vi "MartinsDCtest.vi"() -> ()   [LabVIEW 2011] (continued)
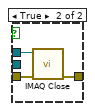
[diagram p3: hidden frame]
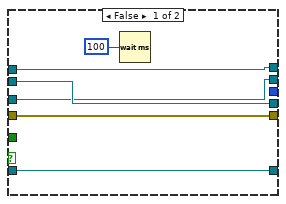
[diagram p5: hidden frame]
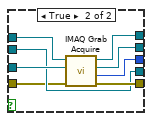
[diagram p6: hidden frame]
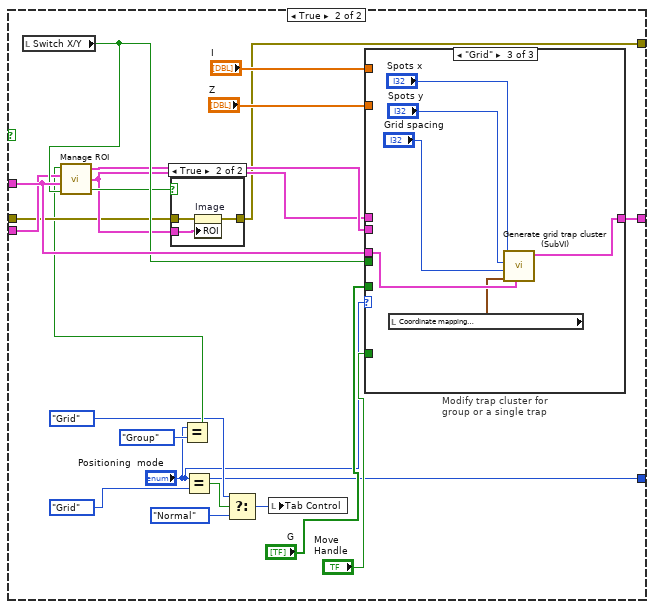
[diagram p11: hidden frame]
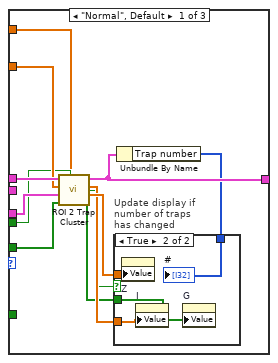
[diagram p13: hidden frame]
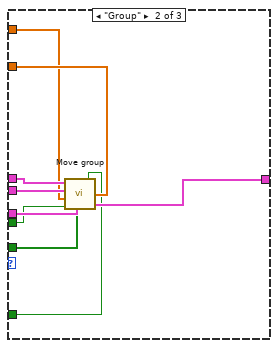
[diagram p15: hidden frame]
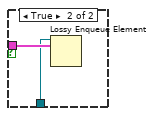
[diagram p17: hidden frame]
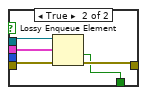
[diagram p19: hidden frame]
        }
      }
      "Step number" <- w131
    }
    n78 = local read "Stop program"() -> (w130:bool)
  }
  n79 = while "User input and events loop" {
    tunnel: w54 -> [w291]
    tunnel: w17 -> [w280]
    tunnel: w19 -> [w279]
    tunnel: w20 -> [w278]
    tunnel: [w277] -> w29
    tunnel: w28 -> [w276]
    tunnel: [w275] -> w27
    stop <- w283 stop-if-true
    w288 = u32 8 items=["Zoom Tool"=8, "Selection Tool"=0, "Pan Tool"=9, "Point Tool"=1, "Line Tool"=2, "Rectangle Tool"=3, "Rotated Rectangle Tool"=12, "Polyline Tool"=10, "Polygon Tool"=5, "Freehand Tool"=11, "Closed Freehand Tool"=6, "Ellipse Tool"=4, "Annulus Tool"=7] ("Current ROI Tool")
    w285 = T10 [enum."LCONTROL"] items=["0", "1", "2", "3", "4", "5", "6", "7", "8", "9", "A", "B", "C", "D", "E", "F", "G", "H", "I", "J", "K", "L", "M", "N", "O", "P", "Q", "R", "S", "T", "U", "V", "W", "X", "Y", "Z", "F1", "F2", "F3", "F4", "F5", "F6", "F7", "F8", "F9", "F10", "F11", "F12", "F13", "F14", "F15", "ADD", "BACK", "BACKSLASH", "CAPITAL", "COMMA", "DECIMAL", "DELETE", "DIVIDE", "DOWN", "END", "EQUALS", "ESCAPE", "GRAVE (`)", "HOME", "INSERT", "LBRACKET", "LCONTROL", "LEFT", "L ALT", "LSHIFT", "LWIN", "MINUS", "MULTIPLY", "NEXT", "NUMLOCK", "NUMPAD_0", "NUMPAD_1", "NUMPAD_2", "NUMPAD_3", "NUMPAD_4", "NUMPAD_5", "NUMPAD_6", "NUMPAD_7", "NUMPAD_8", "NUMPAD_9", "PAUSE", "PERIOD", "PRIOR (PG UP)", "RBRACKET", "RCONTROL", "RETURN", "RIGHT", "R ALT", "RSHIFT", "RWIN", "SCROLL", "SEMICOLON", "SLASH", "SPACE", "SUBTRACT", "TAB", "UP", "ENTER (num pad)", "' (quote)"] ("keys pressed")
    n80 = call-poly <vilib>:"Acquire Input Data.vi"("device ID"=w291, "error in (no error)"=w276) -> ("device ID"=w277:refnum<k1>, "keys pressed"=w284:T10, "error out"=w275:errorcluster)  [unwired: 15 out]
    n81 = property on="Image" class="ImageControl"() -> ("Current ROI Tool"=w287:u32)  [unwired: 2 in, 2 out]
    n82 = Equal?(x=w284, y=w285) -> (x = y?=w286:bool[])
    n83 = Not Equal?(x=w287, y=w288) -> (x != y?=w289:bool)
    n84 = Or Array Elements(Boolean array=w286) -> (logical OR=w290:bool)
    n85 = case shown="True" w289 {
      tunnel: w290 -> [_ w312]
      frame False {
      }
      frame True {
        n86 = case shown="False" w312 {
          frame False {
            w313 = u32 0 items=["Zoom Tool"=8, "Selection Tool"=0, "Pan Tool"=9, "Point Tool"=1, "Line Tool"=2, "Rectangle Tool"=3, "Rotated Rectangle Tool"=12, "Polyline Tool"=10, "Polygon Tool"=5, "Freehand Tool"=11, "Closed Freehand Tool"=6, "Ellipse Tool"=4, "Annulus Tool"=7] ("Current ROI Tool")
            n87 = property on="Image" class="ImageControl"("Current ROI Tool"=w313) -> ()  [unwired: 2 in, 2 out]
          }
          frame True {
            w314 = u32 1 items=["Zoom Tool"=8, "Selection Tool"=0, "Pan Tool"=9, "Point Tool"=1, "Line Tool"=2, "Rectangle Tool"=3, "Rotated Rectangle Tool"=12, "Polyline Tool"=10, "Polygon Tool"=5, "Freehand Tool"=11, "Closed Freehand Tool"=6, "Ellipse Tool"=4, "Annulus Tool"=7] ("Current ROI Tool")
            n88 = property on="Image" class="ImageControl"("Current ROI Tool"=w314) -> ()  [unwired: 2 in, 2 out]
          }
        }
      }
    }
    n89 = Wait (ms)(milliseconds to wait=u32 50) -> ()  [unwired: 1 out]
    n90 = case shown="False" "View Licence" {
      frame False {
      }
      frame True {
        n91 = call "View license.vi"() -> ()  [unwired: 1 in]
      }
    }
    n92 = event shown="[4] \"Image\", \"Positioning  mode\", \"Z\", \"I\", \"Coordinate mapping \n(IMAQ to SLM)\": Mouse Down;  Key Up" {
      selector: _ -> [_ _ _ _ _ _]
      dyn-events: _ -> [_ _ _ _ _ _]
      timeout: 0 -> [_ _ _ _ _ _]
      tunnel: w280 -> [_ _ w302 _ _ _]
      tunnel: w279 -> [_ _ w301 _ _ _]
      tunnel: w278 -> [_ _ w305 _ _ _]
      event Timeout {
        n93 = event-data() -> ()  [unwired: 1 in, 2 out]
      }
      event "Display hologram\nand computed \nimage plane": Value Change {
        n94 = event-data() -> ("NewVal"=w293:bool)  [unwired: 1 in, 4 out]
        n95 = property on="Current trap pos" class="Clust (strict)"("Visible"=w293) -> ()  [unwired: 2 in, 2 out]
        n96 = property on="Displayed Hologram" class="IntGraph (strict)"("Visible"=w293) -> ()  [unwired: 2 in, 2 out]
        n97 = property on="Calculated image plane" class="IntGraph (strict)"("Visible"=w293) -> ()  [unwired: 2 in, 2 out]
        n98 = property on="Property Node" class="VI"() -> ("Front Panel.WinBounds"=w300:T11)  [unwired: 2 in, 2 out]
        n99 = Unbundle By Name(w300) -> ("right"=w299:i16, "left"=w298:i16)
        n100 = Subtract(x=w299, y=w298) -> (x-y=w297:i16)
        n101 = Select(t=i16 500 ("x-y"), s=w293, f=i16 196 ("x-y")) -> (s? t:f=w292:i16)
        n102 = Subtract(x=w297, y=w292) -> (x-y=w296:i16)
        n103 = property on="Splitter" class="Splitter"("Position"=w296) -> ()  [unwired: 2 in, 2 out]
      }
      event "Create path": Value Change {
        n104 = event-data() -> ()  [unwired: 1 in, 5 out]
        n105 = property on="follow path" class="Bool (strict)"("Value"=FALSE) -> ()  [unwired: 2 in, 2 out]
        n106 = Flush Queue "Flush path \nwaypt queue"(queue=w301) -> ()  [unwired: 1 in, 3 out]
        n107 = Preview Queue Element(queue=w302) -> (element=w303:T3, error out=w306:errorcluster)  [unwired: 2 in, 2 out]
        n108 = Flush Queue "Flush path queue"(queue=w305) -> (queue out=w304:refnum<queue>)  [unwired: 1 in, 2 out]
        n109 = Enqueue Element "Enqueue current \ntrap pos in path"(queue=w304, element=w303) -> ()  [unwired: 2 in, 3 out]
        n110 = Enqueue Element "Enqueue current \ntrap pos in path \nwaypts"(queue=w301, element=w303, error in (no error)=w306) -> ()  [unwired: 1 in, 3 out]
      }
      event "cancel path": Value Change {
        n111 = event-data() -> ()  [unwired: 1 in, 5 out]
        n112 = local write "Create path"(FALSE ("Visible")) -> ()
      }
      event "Image", "Positioning  mode", "Z", "I", "Coordinate mapping \n(IMAQ to SLM)": Mouse Down; Key Up {
        n113 = event-data() -> ()  [unwired: 1 in, 3 out]
        n114 = local write "Updating trap cluster"(TRUE ("Update trap positions")) -> ()
      }
      event "Positioning  mode", "Z", "I", "Image", "Coordinate mapping \n(IMAQ to SLM)": Mouse Up {
        n115 = event-data() -> ()  [unwired: 1 in, 7 out]
        n116 = flat-sequence {
          frame #0 {
            n117 = Wait (ms)(milliseconds to wait=u32 100) -> ()  [unwired: 1 out]
          }
          frame #1 {
            n118 = local write "Updating trap cluster"(FALSE ("Update trap positions")) -> ()
          }
        }
      }
    }
    n119 = local read "Stop program"() -> (w283:bool)
  }
  n120 = while "Image acquisition loop" {
    tunnel: w4 -> [w324]
    tunnel: w6 -> [w340]
    tunnel: w8 -> [w339]
    tunnel: [w338] -> w53
    tunnel: [w320] -> w52
    tunnel: w51 -> [w334]
    tunnel: w49 -> [w326]
    shift-right: ["ROI size"] -> _
    shift-left: _ -> [_]
    tunnel: w46 -> [w325]
    tunnel: [w334] -> w44
    tunnel: [w321] -> w43
    tunnel: [w333] -> w42
    tunnel: w7 -> [w332]
    tunnel: w3 -> [w331]
    tunnel: w17 -> [w330]
    tunnel: w20 -> [w329]
    tunnel: w5 -> [w327]
    tunnel: w1 -> [w315]
    stop <- w337 stop-if-true
    n121 = Flush Queue(queue=w325) -> ()  [unwired: 1 in, 3 out]
    n122 = Flush Queue(queue=w326) -> ()  [unwired: 1 in, 3 out]
    n123 = Preview Queue Element(queue=w330, timeout in ms (-1)=10 ("f")) -> (element=w319:T3)  [unwired: 1 in, 3 out]
    n124 = Get Queue Status(queue=w329, return elements? (F)="Display path") -> (elements=w322:T3[])  [unwired: 1 in, 7 out]
    n125 = call <vilib>:"Acquire Semaphore.vi"("semaphore"=w315) -> ("semaphore out"=w317:T9)  [unwired: 4 in, 2 out]
    n126 = case shown="True" w324 {
      tunnel: w340 -> [w345 w357]
      tunnel: w339 -> [w344 w356]
      tunnel: [w344 w355] -> w338
      tunnel: [w343 w354] -> w320
      tunnel: [w345 w353] -> w321
      tunnel: [w346 w352] -> w333
      tunnel: w332 -> [w346 w351]
      tunnel: w331 -> [_ w350]
      tunnel: w327 -> [w343 w349]
      tunnel: [_ w348] -> _
      tunnel: w317 -> [w341 w347]
      tunnel: [w341 w347] -> w316
      frame False {
        n127 = Wait (ms)(milliseconds to wait=u32 100) -> ()  [unwired: 1 out]
      }
      frame True {
        n128 = case shown="True" w350 {
          tunnel: w357 -> [w365 w373]
          tunnel: [w363 w372] -> w355
          tunnel: [w362 w371] -> w354
          tunnel: w356 -> [w363 w370]
          tunnel: [w364 w369] -> w353
          tunnel: [w359 w368] -> w348
          tunnel: [w361 w367] -> w352
          tunnel: w351 -> [w360 w367]
          tunnel: w349 -> [w358 w366]
          frame False {
            n129 = call <vilib>:"IMAQdx Grab.vi"("error in"=w358, "Image In"=w365, "Session In"=w360) -> ("error out"=w362:errorcluster, "Buffer Number Out"=w359:u32, "Image Out"=w364:T2, "Session Out"=w361:T7)  [unwired: 5 in]
          }
          frame True {
            n130 = call <vilib>:"IMAQ Grab Acquire.vi"("error in (no error)"=w366, "Image In"=w373, "IMAQ Session In"=w370) -> ("error out"=w371:errorcluster, "Acquired Buffer Number"=w368:u32, "Image Out"=w369:T2, "IMAQ Session Out"=w372:refnum<k11>)  [unwired: 1 in, 4 out]
          }
        }
      }
    }
    n131 = call "Create trap overlay.vi"("Current trap cluster"=w319, "Image in"=w321, "ROI size"="ROI size", "Switch X/Y"="Switch X/Y", "Path"=w322) -> ()  [unwired: 1 out]
    n132 = case shown="True" "Show image" {
      tunnel: w321 -> [_ w374]
      frame False {
      }
      frame True {
        "Image" <- w374
      }
    }
    n133 = call <vilib>:"Release Semaphore.vi"("semaphore"=w316) -> ()  [unwired: 5 in, 2 out]
    n134 = local read "Stop program"() -> (w337:bool)
  }
  n135 = while "Trap position loop" {
    tunnel: w19 -> [w386]
    tunnel: w20 -> [w383]
    shift-right: [w385] -> _
    shift-left: w16 -> [w378]
    tunnel: w18 -> [w384]
    tunnel: w17 -> [w381]
    tunnel: [w380] -> w35
    tunnel: w21 -> [w377]
    tunnel: [w375] -> w33
    stop <- "Stop program" stop-if-true
    n136 = property on="Image" class="ImageControl"(error in=w377) -> (error out=w376:errorcluster, "ROI"=w380:T1)  [unwired: 1 in, 1 out]
    n137 = case shown="False" "Run calibration" {
      selector: "Run calibration" -> [_ w582]
      tunnel: w386 -> [w411 _]
      tunnel: w378 -> [w410 w581]
      tunnel: [w390 w581] -> w385
      tunnel: w384 -> [w401 w591]
      tunnel: w383 -> [w399 _]
      tunnel: w381 -> [w396 _]
      tunnel: w380 -> [w395 w590]
      tunnel: w376 -> [w394 w586]
      tunnel: [w392 w583] -> w375
      frame False {
        n138 = case "Update trap cluster" shown="False" "Updating trap cluster" {
          tunnel: w410 -> [w413 w434]
          tunnel: [w413 w427] -> w402
          tunnel: w395 -> [_ w425]
          tunnel: w394 -> [w412 w424]
          tunnel: [w412 w423] -> w393
          tunnel: [_ "Positioning  mode"] -> w387
          frame False {
          }
          frame True {
            n139 = local read "Switch X/Y"() -> (w433:bool)
            n140 = Equal?(x="Positioning  mode", y=enum16{"Normal", "Group", "Grid"}."Group") -> (x = y?=w421:bool)
            n141 = call "Manage ROI.vi"("Switch X/Y"=w433, "Trap cluster in"=w434, "ROI in"=w425, "Group traps"=w421) -> ("Replace ROI"=w432:bool, "ROI out"=w426:T1, "Previous ROI out"=w431:T1)
            n142 = case shown="True" w432 {
              tunnel: w426 -> [_ w438]
              tunnel: w424 -> [w435 w437]
              tunnel: [w435 w436] -> w423
              frame False {
              }
              frame True {
                n143 = property on="Image" class="ImageControl"(error in=w437, "ROI"=w438) -> (error out=w436:errorcluster)  [unwired: 1 in, 1 out]
              }
            }
            n144 = Equal?(x="Positioning  mode", y=enum16{"Normal", "Group", "Grid"}."Grid") -> (x = y?=w419:bool)
            n145 = Select(t=enum32{"Normal", "Grid"}."Grid", s=w419, f=enum32{"Normal", "Grid"}."Normal" ("Tab Control")) -> (s? t:f=w416:enum32{"Normal", "Grid"})
            n146 = local write "Tab Control"(w416) -> ()
            n147 = case "Modify trap cluster for \ngroup or a single trap" shown="\"Grid\"" "Positioning  mode" {
              tunnel: [w443 w460 w465] -> w427
              tunnel: w426 -> [w450 w461 _]
              tunnel: w434 -> [w449 w463 w466]
              tunnel: w431 -> [_ w462 _]
              tunnel: "Z" -> [w448 w459 _]
              tunnel: "Move \nHandle" -> [_ w458 _]
              tunnel: w433 -> [w447 w457 _]
              tunnel: "I" -> [w445 w456 _]
              tunnel: "G" -> [w440 w455 _]
              frame "Normal", Default {
                n148 = call "ROI 2 Trap Cluster.vi"("Amplitudes"=w445, "Switch X/Y"=w447, "Group"=w440, "Trap Cluster in"=w449, "Z"=w448, "ROI"=w450) -> ("Group out"=w439:bool[], "Z out"=w446:dbl[], "Amplitudes out"=w444:dbl[], "Trap Cluster Out"=w443:T3, "Update display"=w441:bool)
                n149 = Unbundle By Name(w443) -> ("Trap number"=w442:i32[])
                n150 = case "Update display if\nnumber of traps \nhas changed" shown="True" w441 {
                  tunnel: w446 -> [_ w454]
                  tunnel: w444 -> [_ w453]
                  tunnel: w442 -> [_ w452]
                  tunnel: w439 -> [_ w451]
                  frame False {
                  }
                  frame True {
                    n151 = property on="Z" class="Arr (strict)"("Value"=w454) -> ()  [unwired: 2 in, 2 out]
                    n152 = property on="I" class="Arr (strict)"("Value"=w453) -> ()  [unwired: 2 in, 2 out]
                    n153 = property on="G" class="Arr (strict)"("Value"=w451) -> ()  [unwired: 2 in, 2 out]
                    "#" <- w452
                  }
                }
              }
              frame "Group" {
                n154 = call "Move group.vi"("New handle position in"=w461, "Trap cluster in"=w463, "Previous handle position in"=w462, "Amplitudes"=w456, "Group"=w455, "Switch X/Y"=w457, "Move handle"=w458, "Z"=w459) -> ("Trap cluster out"=w460:T3)
              }
              frame "Grid" {
                n155 = local read "Coordinate mapping \n(IMAQ to SLM)"() -> (w464:T5)
                n156 = call "Generate grid trap cluster (SubVI).vi"("output cluster 3"=w466, "Coordinate mapping \n(IMAQ to SLM)"=w464, "Grid spacing"="Grid spacing", "Spots y"="Spots y", "Spots x"="Spots x") -> ("output cluster 2"=w465:T3)  [unwired: 6 in]
              }
            }
          }
        }
        n157 = Wait (ms)(milliseconds to wait=u32 50) -> ()  [unwired: 1 out]
        n158 = Unbundle By Name("Path controls") -> ("Add current \npositions to path"=w397:bool, "Synchronize traps"=w406:bool, "Step length"=w388:dbl, "follow path"=w400:bool, "Arrive \nsimultaneously"=w408:bool)
        n159 = Or(x=w397, y=w406) -> (x .or. y?=w407:bool)
        n160 = Or(x=w406, y=w400) -> (x .or. y?=w404:bool)
        n161 = Or(x=w407, y=w400) -> (x .or. y?=w405:bool)
        n162 = case shown="True" "Create path" {
          tunnel: w411 -> [_ w484]
          tunnel: w402 -> [w470 w478]
          tunnel: w388 -> [_ w492]
          tunnel: w399 -> [_ w488]
          tunnel: w408 -> [_ w491]
          tunnel: w405 -> [_ w490]
          tunnel: w404 -> [_ w489]
          tunnel: w400 -> [_ w477]
          tunnel: w401 -> [w473 w485]
          tunnel: w396 -> [_ w483]
          tunnel: w395 -> [_ w482]
          tunnel: w393 -> [w472 w481]
          tunnel: [w472 w480] -> w392
          tunnel: "Updating trap cluster" -> [w471 _]
          tunnel: [w470 w479] -> w390
          tunnel: w387 -> [_ w476]
          frame False {
            n163 = case shown="False" w471 {
              tunnel: w470 -> [_ w475]
              tunnel: w473 -> [_ w474]
              frame False {
              }
              frame True {
                n164 = Lossy Enqueue Element(queue=w474, element=w475) -> ()  [unwired: 1 in, 4 out]
              }
            }
          }
          frame True {
            n165 = Lossy Enqueue Element "Enqueue\noverlay pos"(queue=w483, element=w478) -> ()  [unwired: 1 in, 4 out]
            n166 = case "Add wpt" shown="True" w490 {
              tunnel: w478 -> [_ w572]
              tunnel: w484 -> [w569 w573]
              tunnel: [w569 w570] -> w493
              tunnel: [_ w571] -> w486
              frame False {
              }
              frame True {
                n167 = Enqueue Element "Enqueue path\n waypts"(queue=w573, element=w572) -> (queue out=w570:refnum<queue>, error out=w571:errorcluster)  [unwired: 2 in, 1 out]
              }
            }
            n168 = case "Compute path" shown="True" w489 {
              tunnel: w493 -> [_ w580]
              tunnel: w488 -> [_ w579]
              tunnel: w492 -> [_ w578]
              tunnel: w491 -> [_ w577]
              tunnel: [w574 w575] -> w487
              tunnel: w486 -> [w574 w576]
              frame False {
              }
              frame True {
                n169 = call "compute path cluster.vi"("path queue"=w579, "Arrive simultaeously"=w577, "error in (no error)"=w576, "Step length\n(IMAQ pixels)"=w578, "waypoint queue"=w580) -> ("error out"=w575:errorcluster)  [unwired: 2 in]
              }
            }
            n170 = case "Follow path" shown="True" w477 {
              tunnel: w488 -> [_ w524]
              tunnel: w487 -> [_ w525]
              tunnel: w485 -> [_ w527]
              tunnel: w484 -> [_ w526]
              tunnel: w482 -> [_ w523]
              tunnel: w481 -> [w495 w504]
              tunnel: [w495 w503] -> w480
              tunnel: [w494 w498] -> w479
              tunnel: w478 -> [w494 _]
              tunnel: w476 -> [_ w497]
              frame False {
              }
              frame True {
                w518 = TRUE ("Visible")
                n171 = Flush Queue "Flush Waypts"(queue=w526, error in (no error)=w525) -> (error out=w517:errorcluster)  [unwired: 2 out]
                n172 = Get Queue Status(queue=w524, error in (no error)=w517) -> (queue out=w521:refnum<queue>, error out=w516:errorcluster, # elements in queue=w520:i32)  [unwired: 1 in, 5 out]
                n173 = property on="Pause" class="Bool (strict)"(error in=w516, "Visible"=w518) -> (error out=w515:errorcluster)  [unwired: 1 in, 1 out]
                n174 = property on="cancel path" class="Bool"(error in=w515, "Visible"=w518) -> (error out=w514:errorcluster)  [unwired: 1 in, 1 out]
                n175 = for {
                  N: w520 -> [_]
                  tunnel: w514 -> [w547]
                  tunnel: w527 -> [w549]
                  tunnel: w521 -> [w545]
                  tunnel: [w545] -> w519
                  tunnel: [FALSE ("Group traps")] -> w499
                  shift-right: [w536] -> w498
                  shift-left: _ -> [w538]
                  tunnel: [w535] -> w513
                  tunnel: [w532] -> w511 mode=indexing
                  tunnel: [w533] -> w507
                  tunnel: [TRUE ("Display path")] -> w505
                  tunnel: w497 -> [_]
                  tunnel: "Step time \n(ms)" -> [w528]
                  i -> [w533]
                  stop <- w542 stop-if-true
                  n176 = Dequeue Element(queue=w545, timeout in ms (-1)=0, error in (no error)=w547) -> (element=w537:T3, timed out?=w541:bool, error out=w548:errorcluster)  [unwired: 1 out]
                  n177 = while {
                    tunnel: [w566] -> w539
                    tunnel: ["cancel path"] -> w534
                    tunnel: w528 -> [w563]
                    stop <- w568 stop-if-true
                    n178 = local read "Stop program"() -> (w566:bool)
                    n179 = Wait (ms)(milliseconds to wait=w563) -> ()  [unwired: 1 out]
                    n180 = Or(x=w566, y="cancel path") -> (x .or. y?=w564:bool)
                    n181 = Implies(1:w564, 2:"Pause") -> (0:w568:bool)
                  }
                  n182 = case shown="False" "Skip step if \ntimed out" {
                    tunnel: w549 -> [w555 w560]
                    tunnel: w548 -> [w554 w558]
                    tunnel: [FALSE ("overflow?") w556] -> w540
                    tunnel: w537 -> [w553 w559]
                    tunnel: [w552 w557] -> w535
                    tunnel: 2000 ("timeout in ms (-1)") -> [w551 _]
                    frame False {
                      n183 = Enqueue Element "Enqueue trap pos"(queue=w555, element=w553, timeout in ms (-1)=w551, error in (no error)=w554) -> (error out=w552:errorcluster)  [unwired: 2 out]
                    }
                    frame True {
                      n184 = Lossy Enqueue Element(queue=w560, element=w559, error in (no error)=w558) -> (overflow?=w556:bool, error out=w557:errorcluster)  [unwired: 2 out]
                    }
                  }
                  "Step skipped" <- w540
                  n185 = case shown="False" w539 {
                    tunnel: w538 -> [_ w562]
                    tunnel: w537 -> [w561 _]
                    tunnel: [w561 w562] -> w536
                    frame False {
                    }
                    frame True {
                    }
                  }
                  n186 = Or(x=w534, y=w539) -> (x .or. y?=w544:bool)
                  n187 = Or(x=w544, y=w541) -> (x .or. y?=w542:bool)
                  n188 = Tick Count (ms)() -> (millisecond timer value=w532:u32)
                }
                n189 = local write "Display path"(FALSE ("Display path")) -> ()
                n190 = local read "Switch X/Y"() -> (w501:bool)
                n191 = call "Trap cluster 2 ROI.vi"("Switch X/Y"=w501, "Trap cluster"=w498, "ROI in"=w523) -> ("ROI out"=w522:T1)
                n192 = local write "Positioning  mode"(w497) -> ()
                n193 = local write "Step skipped"(w499) -> ()
                n194 = local write "Create path"(w499) -> ()
                n195 = local write "Display path"(w505) -> ()
                n196 = property on="Pause" class="Bool (strict)"(error in=w513, "Visible"=w499, "Value"=w499) -> (error out=w512:errorcluster)  [unwired: 1 in, 1 out]
                n197 = property on="cancel path" class="Bool"(error in=w512, "Visible"=w499) -> ()  [unwired: 1 in, 2 out]
                n198 = property on="Image" class="ImageControl"(error in=w504, "ROI"=w522) -> (error out=w503:errorcluster)  [unwired: 1 in, 1 out]
                n199 = property on="follow path" class="Bool (strict)"("Value"=w499) -> ()  [unwired: 2 in, 2 out]
                n200 = Array Max & Min(array=w511) -> (max value=w510:u32, min value=w509:u32)  [unwired: 2 out]
                n201 = Subtract(x=w510, y=w509) -> (x-y=w508:u32)
                n202 = Increment(x=w507) -> (x+1=w502:i32)
                n203 = Divide(x=w508, y=w502) -> (x/y=→"Average step time (ms)":dbl)
                n204 = Flush Queue "Flush Path"(queue=w519) -> ()  [unwired: 1 in, 3 out]
              }
            }
          }
        }
        n205 = case shown="True" "Apply Corrections" {
          frame False {
          }
          frame True {
            n206 = call "Apply Corrections.vi"() -> ()  [unwired: 1 in]
          }
        }
      }
      frame True {
        n207 = property on="Cancel calibration" class="Bool"("Visible"=w582) -> ()  [unwired: 2 in, 2 out]
        n208 = local read "Coordinate mapping \n(IMAQ to SLM)"() -> (w589:T5)
        n209 = flat-sequence {
          tunnel: [w605] -> w595
          tunnel: [w607] -> w594
          tunnel: w590 -> [w605]
          tunnel: w589 -> [w599]
          tunnel: [w596] -> w588
          tunnel: [w599] -> w587
          tunnel: w586 -> [w598]
          tunnel: [w597] -> w584
          tunnel: [w620] -> w593
          tunnel: w595 -> [w620]
          tunnel: w594 -> [w614]
          tunnel: [w616] -> w592
          tunnel: w591 -> [w619]
          tunnel: w588 -> [w618]
          tunnel: w587 -> [w615]
          tunnel: [w612] -> w585
          tunnel: w584 -> [w612]
          tunnel: w593 -> [w675]
          tunnel: w585 -> [w673]
          tunnel: [w672] -> w583
          frame #0 {
            w608 = u32 8 items=["Zoom Tool"=8, "Selection Tool"=0, "Pan Tool"=9, "Point Tool"=1, "Line Tool"=2, "Rectangle Tool"=3, "Rotated Rectangle Tool"=12, "Polyline Tool"=10, "Polygon Tool"=5, "Freehand Tool"=11, "Closed Freehand Tool"=6, "Ellipse Tool"=4, "Annulus Tool"=7] ("Current ROI Tool")
            n210 = Bundle By Name(cluster=w599, "sX"=0.0, "sY"=0.0, "cX"=1.0 ("sX"), "cY"=1.0) -> (w596:T5)
            n211 = local write "Coordinate mapping \n(IMAQ to SLM)"(w596) -> ()
            n212 = property on="ok" class="Bool"("Visible"=TRUE ("ROI Tool Buttons Visibile:Zoom Tool Button Visible")) -> ()  [unwired: 2 in, 2 out]
            n213 = property on="Image" class="ImageControl"("Current ROI Tool"=w608) -> ()  [unwired: 2 in, 2 out]
            n214 = Two Button Dialog(message="Mark the center of the \ndisplayed spot using the \nzoom and the point tool, \nthen click the OK button. \n(Will be repeated three times)", 1:"Cancel" ("F button name (\"Cancel\")"), 2:"Start calibration" ("T button name (\"OK\")")) -> (T button?=w607:bool)
            n215 = property on="Image" class="ImageControl"(error in=w598, "ROI"=T1 {"Global Rectangle"=[100, 100, 394, 354], "Contours"=[{"Contour Type"=0, "ROI Type"=1, "Points"=[100, 100]}]} ("ROI 2")) -> (error out=w597:errorcluster)  [unwired: 1 in, 1 out]
          }
          frame #1 {
            n216 = case shown="True" w614 {
              tunnel: w618 -> [w624 w635]
              tunnel: [w624 w630] -> w617
              tunnel: w619 -> [_ w626]
              tunnel: [TRUE ("Stop program") w625] -> w613
              frame False {
              }
              frame True {
                n217 = for {
                  tunnel: [w662] -> w644 mode=indexing
                  tunnel: [w661] -> w643 mode=indexing
                  tunnel: T3[] [{"X (IMAQ)"=[-64.0], "Y (IMAQ)"=[-64.0], "Z"=[0.0], "Amplitudes"=[1.0], "Trap number"=[0], "ROI number"=[0], "Number of traps"=1, "Group"=[]}, {"X (IMAQ)"=[64.0], "Y (IMAQ)"=[-64.0], "Z"=[0.0], "Amplitudes"=[1.0], "Trap number"=[0], "ROI number"=[0], "Number of traps"=1, "Group"=[]}, {"X (IMAQ)"=[-64.0], "Y (IMAQ)"=[64.0], "Z"=[0.0], "Amplitudes"=[1.0], "Trap number"=[0], "ROI number"=[0], "Number of traps"=0, "Group"=[]}] -> [w659] mode=indexing
                  tunnel: [w656] -> w628 mode=indexing
                  tunnel: [w654] -> w627 mode=indexing
                  tunnel: w626 -> [w658]
                  tunnel: [w653] -> w625
                  stop <- w653 stop-if-true
                  n218 = while {
                    tunnel: [w669] -> w660
                    tunnel: [w665] -> w653
                    stop <- w667 stop-if-true
                    n219 = local read "Stop program"() -> (w666:bool)
                    n220 = Wait (ms)(milliseconds to wait=u32 50) -> ()  [unwired: 1 out]
                    n221 = Or(x=w666, y="Cancel calibration") -> (x .or. y?=w665:bool)
                    n222 = property on="Image" class="ImageControl"() -> ("ROI"=w669:T1)  [unwired: 2 in, 2 out]
                    n223 = Or(x="ok", y=w665) -> (x .or. y?=w667:bool)
                  }
                  n224 = Enqueue Element "Enqueue trap pos"(queue=w658, element=w659) -> ()  [unwired: 2 in, 3 out]
                  n225 = Unbundle By Name(w660) -> ("Global Rectangle"=w663:i32[])  [unwired: 1 out]
                  n226 = Unbundle By Name(w659) -> ("X (IMAQ)"=w657:dbl[], "Y (IMAQ)"=w655:dbl[])
                  n227 = Index Array(array=w657) -> (element=w656:dbl)  [unwired: 1 in]
                  n228 = Index Array(array=w655) -> (element=w654:dbl)  [unwired: 1 in]
                  n229 = Index Array(array=w663) -> (element #1=w662:i32, element #2=w661:i32)  [unwired: 2 in]
                }
                n230 = Index Array(array=w643) -> (element #1=w645:i32, element #2=w646:i32)  [unwired: 2 in]
                n231 = Index Array(array=w644) -> (element #1=w647:i32, element #2=w648:i32)  [unwired: 2 in]
                n232 = Subtract(x=w648, y=w647) -> (x-y=w640:i32)
                n233 = Subtract(x=w646, y=w645) -> (x-y=w638:i32)
                n234 = Absolute Value(x=w638) -> (abs(x)=w637:i32)
                n235 = Absolute Value(x=w640) -> (abs(x)=w639:i32)
                n236 = Less?(x=w639, y=w637) -> (x < y?=w636:bool)
                n237 = case shown="False" w636 {
                  tunnel: w644 -> [w650 w652]
                  tunnel: w643 -> [w649 w651]
                  tunnel: [w649 w652] -> w641
                  tunnel: [w650 w651] -> w642
                  frame False {
                  }
                  frame True {
                  }
                }
                n238 = formula code="cX = (xSLM[1] - xSLM[0]) / (xIMAQ[1] - xIMAQ[0]); \ncY = (ySLM[2] - ySLM[0]) / (yIMAQ[2] - yIMAQ[0]); \n\nsX = xSLM[0] - xIMAQ[0] *cX;\nsY = ySLM[0] - yIMAQ[0] *cY;"("xIMAQ"=w642, "yIMAQ"=w641, "xSLM"=w628, "ySLM"=w627) -> ("cX"=w634:dbl, "cY"=w633:dbl, "sX"=w632:dbl, "sY"=w631:dbl)
                n239 = property on="Switch X/Y" class="Bool (strict)"("Value"=w636) -> ()  [unwired: 2 in, 2 out]
                n240 = Bundle By Name(cluster=w635, "cX"=w634, "cY"=w633, "sX"=w632, "sY"=w631) -> (w630:T5)
              }
            }
            n241 = case "Calibration canceled?" shown="True" w613 {
              tunnel: w617 -> [w621 _]
              tunnel: [w621 w622] -> w616
              tunnel: w615 -> [_ w622]
              frame False {
              }
              frame True {
              }
            }
          }
          frame #2 {
            w671 = FALSE ("ROI Tool Buttons Visibile:Zoom Tool Button Visible")
            w674 = u32 1 items=["Zoom Tool"=8, "Selection Tool"=0, "Pan Tool"=9, "Point Tool"=1, "Line Tool"=2, "Rectangle Tool"=3, "Rotated Rectangle Tool"=12, "Polyline Tool"=10, "Polygon Tool"=5, "Freehand Tool"=11, "Closed Freehand Tool"=6, "Ellipse Tool"=4, "Annulus Tool"=7] ("Current ROI Tool")
            n242 = property on="Image" class="ImageControl"(error in=w673, "ROI"=w675) -> (error out=w672:errorcluster)  [unwired: 1 in, 1 out]
            n243 = property on="Image" class="ImageControl"("Current ROI Tool"=w674, "Point Tool Button Visibile"=w671) -> ()  [unwired: 2 in, 2 out]
            n244 = property on="Cancel" class="Bool"("Visible"=w671) -> ()  [unwired: 2 in, 2 out]
            n245 = property on="ok" class="Bool"("Visible"=w671) -> ()  [unwired: 2 in, 2 out]
          }
        }
        n246 = local write "Coordinate mapping \n(IMAQ to SLM)"(w592) -> ()
      }
    }
  }
  n247 = property on="Show image" class="Bool (strict)"("Visible"=w41) -> ()  [unwired: 2 in, 2 out]
  n248 = property on="ROI size" class="DigNum (strict)"("Visible"=w41) -> ()  [unwired: 2 in, 2 out]
  n249 = property on="Measure" class="Bool"("Visible"=w41) -> ()  [unwired: 2 in, 2 out]
  n250 = call-poly <vilib>:"Close Input Device.vi"("error in (no error)"=w27, "device ID"=w29) -> ()  [unwired: 9 out]
  n251 = call "FreeGPUandSLM.vi"("error in"=w32) -> ("error out"=w31:errorcluster)  [unwired: 1 out]
  "CUDA/SLM error" <- w31
  n252 = case shown="True" w4 {
    tunnel: w53 -> [_ w681]
    tunnel: w52 -> [w676 w680]
    tunnel: w42 -> [_ w679]
    tunnel: w3 -> [_ w678]
    tunnel: [w676 w677] -> w34
    frame False {
    }
    frame True {
      n253 = case shown="False" w678 {
        tunnel: w681 -> [_ w687]
        tunnel: w680 -> [w684 w686]
        tunnel: [w683 w685] -> w677
        tunnel: w679 -> [w682 _]
        frame False {
          n254 = call <vilib>:"IMAQdx Close Camera.vi"("error in"=w684, "Session In"=w682) -> ("error out"=w683:errorcluster)  [unwired: 9 in]
        }
        frame True {
          n255 = call <vilib>:"IMAQ Close.vi"("error in (no error)"=w686, "IMAQ Session In"=w687) -> ("error out"=w685:errorcluster)  [unwired: 9 in]
        }
      }
    }
  }
  n256 = Merge Errors(w34, w33) -> (w30:errorcluster)
  "NI Vision error" <- w30
  n257 = call "IMAQ Dispose"("Image"=w43) -> ()  [unwired: 5 in, 1 out]
  n258 = for {
    tunnel: w44 -> [w688] mode=indexing
    n259 = call "IMAQ Dispose"("Image"=w688) -> ()  [unwired: 5 in, 1 out]
  }
  n260 = Unbundle By Name(w35) -> ("Contours"=w40:T12)
  n261 = Index Array(array=w40) -> (element=w39:T13)  [unwired: 1 in]
  n262 = flat-sequence {
    tunnel: w31 -> [_]
    tunnel: w30 -> [_]
    frame #0 {
      n263 = local write "Stop program"(FALSE ("Stop program")) -> ()
    }
  }
  n264 = Unbundle By Name(w39) -> ("ROI Type"=w38:u32)
  n265 = Equal?(x=w38, y=u32 1) -> (x = y?=w36:bool)
  n266 = case shown="True" w36 {
    tunnel: w35 -> [_ w690]
    frame False {
    }
    frame True {
      n267 = local write "ROI"(w690) -> ()
    }
  }
